vi "Main.vi"() -> ()   [LabVIEW 2020]
uses:
  SET-.ctl
  SET+.ctl
  indicater_CRUI_setpooint.ctl
  I1.ctl
  DIS.ctl
  CRUIONOFF.ctl
  CRUISEVOLUM.ctl
  THONG/STOP.ctl
  CHARDC.ctl
  <vilib>/addons/control/pid/autopid.llb/PID autotuning parameters (adv).ctl
  BRAKE.ctl
  GAS.ctl
  ODOVELICOCITY.ctl
  RPM.ctl
  indicater_dis.ctl
  indicater_Time.ctl
  indicater_taget.ctl
  <vilib>/addons/control/pid/pid.llb/PID Time Unit.ctl
  <vilib>/addons/control/pid/pid.llb/PID Structure.ctl
  <vilib>/addons/control/pid/pid.llb/PID Gain Unit.ctl
  LITMIT.ctl
  SETLIMIT+.ctl
  SETLIMIT-.ctl
  indicater_lit.ctl
  indicater_PWM.ctl
  P.ctl
  R.ctl
  N.ctl
  D.ctl
  CCC.ctl
  <vilib>/Instr/_visa.llb/VISA Configure Serial Port (Instr).vi
  <vilib>/addons/control/pid/pid.llb/PID Structure Conversion (DBL).vi
  <vilib>/addons/control/pid/pid.llb/PID Advanced (DBL).vi
  <vilib>/addons/control/pid/NI_PID_autopid.lvlib
  <vilib>/ptbypt/NI_PtbyPt.lvlib
  <vilib>/addons/control/pid/NI_PID_pid.lvlib
panel:
  out "Waveform Chart 2":T1
  out "D":T2
  out "N":T3
  out "R":T4
  out "P":T5=TRUE
  out "PWM Previous":T6
  in  "auto? ACC":bool
  out "Limit Setpoint":T7
  out "Limit Active":bool
  in  "Limit -":T8
  in  "Limit +":T9
  in  "Limit Speed":T10
  in  "gamma":dbl format="%.2f"
  in  "alpha":dbl=0.2 format="%.2f"
  in  "CHARDC.ctlproportional unit":T11 items=["Gain (K)", "Band (PB)"]
  in  "PID structure":T12 items=["Academic (Standard)", "Parallel", "Series"]
  in  "derivative unit":T13=1 items=["min", "s"]
  in  "integral unit":T13=1 items=["min", "s"]
  in  "derivative":dbl
  in  "integral":dbl
  in  "proportional":dbl=10.0
  in  "linearity":dbl=0.9 format="%.2f"
  in  "beta":dbl=0.7 format="%.2f"
  in  "reinitialize? (F) 2":bool
  out "Speed Setpoint (km/h)":dbl
  out "Target Distance (m)":T14
  out "Time Level":T15=1
  out "Distance (m)":T16=53
  out "Brake Light":bool
  in  "VISA resource name":refnum<visa-resource-name>="COM15"
  in  "baud rate":u32=115200
  out "RPM":T17 scale=0.0..650.0
  out "VELOCITY":T18 scale=0.0..250.0
  out "GAS PEDAL":T19 scale=0.0..700.0
  out "BRAKE PEDAL":T20=1 scale=0.0..700.0
  in  "autotune? (F)":bool
  in  "PID gains":T21={"proportional gain (Kc)"=0.261831, "integral time (Ti, min)"=0.013639, "derivative time (Td, min)"=0.0} {"derivative time (Td, min)" format="%#.6g"; "integral time (Ti, min)" format="%#.6g"; "proportional gain (Kc)" format="%#.6g"}
  in  "dt (s)":dbl=0.02
  in  "reinitialize? (F)":bool
  in  "autotuning parameters":T22={"technique"=0, "type of controller"=1, "control specification"=0, "amplitude"=30.0} {"amplitude" format="%.2f"; "control specification" items=["normal", "fast", "slow"]; "type of controller" items=["P", "PI", "PID"]; "technique" items=["Step Open Loop", "Step Closed Loop", "Relay", "PID Relay"]}
  out "completed?":bool
  out "tuned PID gains":T23={"proportional gain (Kc)"=0.638776, "CHARDC.ctlintegral time (Ti, min)"=0.011721, "derivative time (Td, min)"=0.0} {"derivative time (Td, min)" format="%#.6g"; "CHARDC.ctlintegral time (Ti, min)" format="%#.6g"; "proportional gain (Kc)" format="%#.6g"}
  in  "auto? Speed Control":bool
  in  "ACCEPT SPEED PID":bool
  out "MOTOR CONTROL":T24
  in  "stop":T25
  in  "PID Mode":T26=1 scale=1.0..3.0
  in  "Cruise Enable":T27
  in  "Distance":T28
  out "Distance Level":T29=1
  out "Cruise Active":bool
  out "Cruise Setpoint":T30
  in  "Speed +":T31
  in  "Speed -":T32
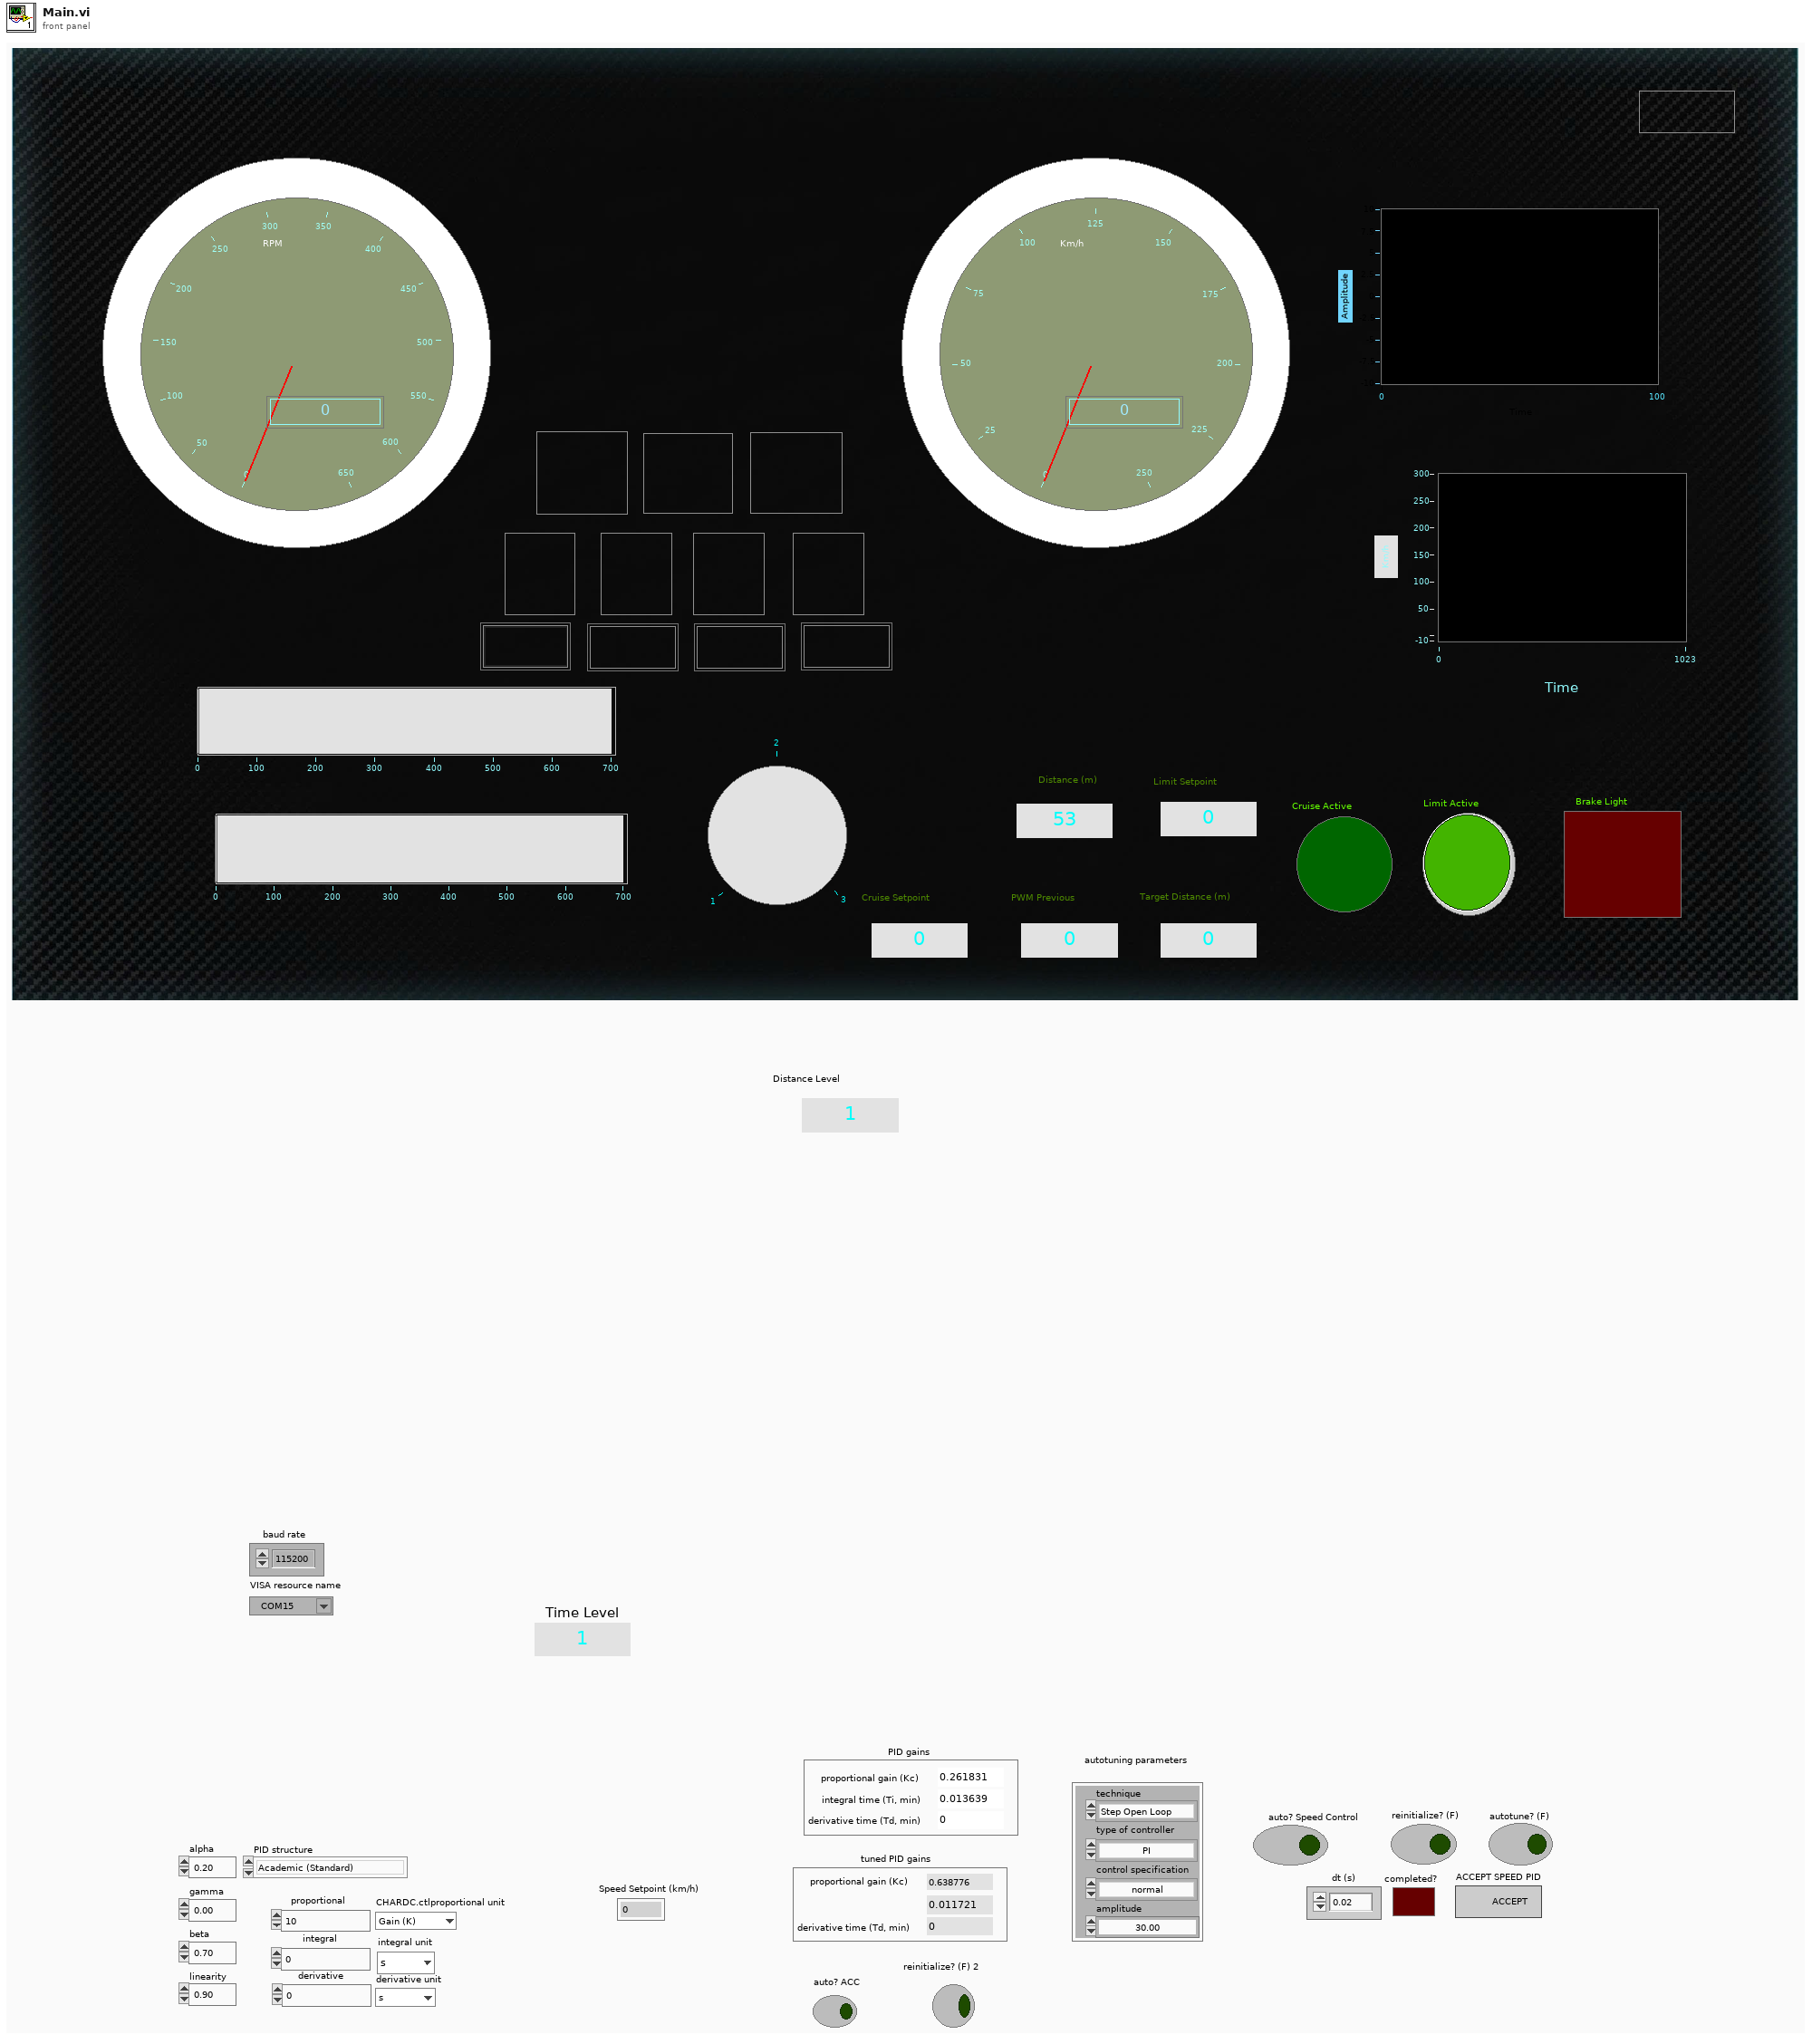
[diagram p1: front panel]
types:
  T1 = typedef "CCC.ctl" = cluster{"VELOCITY":u16, "Cruise Setpoint":u64}
  T2 = typedef "D.ctl" = bool
  T3 = typedef "N.ctl" = bool
  T4 = typedef "R.ctl" = bool
  T5 = typedef "P.ctl" = bool
  T6 = typedef "indicater_PWM.ctl" = i8
  T7 = typedef "indicater_lit.ctl" = i8
  T8 = typedef "SETLIMIT-.ctl" = bool
  T9 = typedef "SETLIMIT+.ctl" = bool
  T10 = typedef "LITMIT.ctl" = bool
  T11 = typedef "NI_PID_pid.lvlib/PID Gain Unit.ctl" = u16
  T12 = typedef "NI_PID_pid.lvlib/PID Structure.ctl" = u16
  T13 = typedef "NI_PID_pid.lvlib/PID Time Unit.ctl" = u16
  T14 = typedef "indicater_taget.ctl" = i8
  T15 = typedef "indicater_Time.ctl" = i8
  T16 = typedef "indicater_dis.ctl" = i8
  T17 = typedef "RPM.ctl" = u16
  T18 = typedef "ODOVELICOCITY.ctl" = u16
  T19 = typedef "GAS.ctl" = u8
  T20 = typedef "BRAKE.ctl" = u8
  T21 = cluster{"proportional gain (Kc)":dbl, "integral time (Ti, min)":dbl, "derivative time (Td, min)":dbl}
  T22 = typedef "NI_PID_autopid.lvlib/PID autotuning parameters (adv).ctl" = cluster{"technique":u16, "type of controller":u16, "control specification":u16, "amplitude":dbl}
  T23 = cluster{"proportional gain (Kc)":dbl, "CHARDC.ctlintegral time (Ti, min)":dbl, "derivative time (Td, min)":dbl}
  T24 = typedef "CHARDC.ctl" = dbl
  T25 = typedef "STOP.ctl" = bool
  T26 = typedef "CRUISEVOLUM.ctl" = u8
  T27 = typedef "CRUIONOFF.ctl" = bool
  T28 = typedef "DIS.ctl" = bool
  T29 = typedef "I1.ctl" = i8
  T30 = typedef "indicater_CRUI_setpooint.ctl" = i8
  T31 = typedef "SET+.ctl" = bool
  T32 = typedef "SET-.ctl" = bool
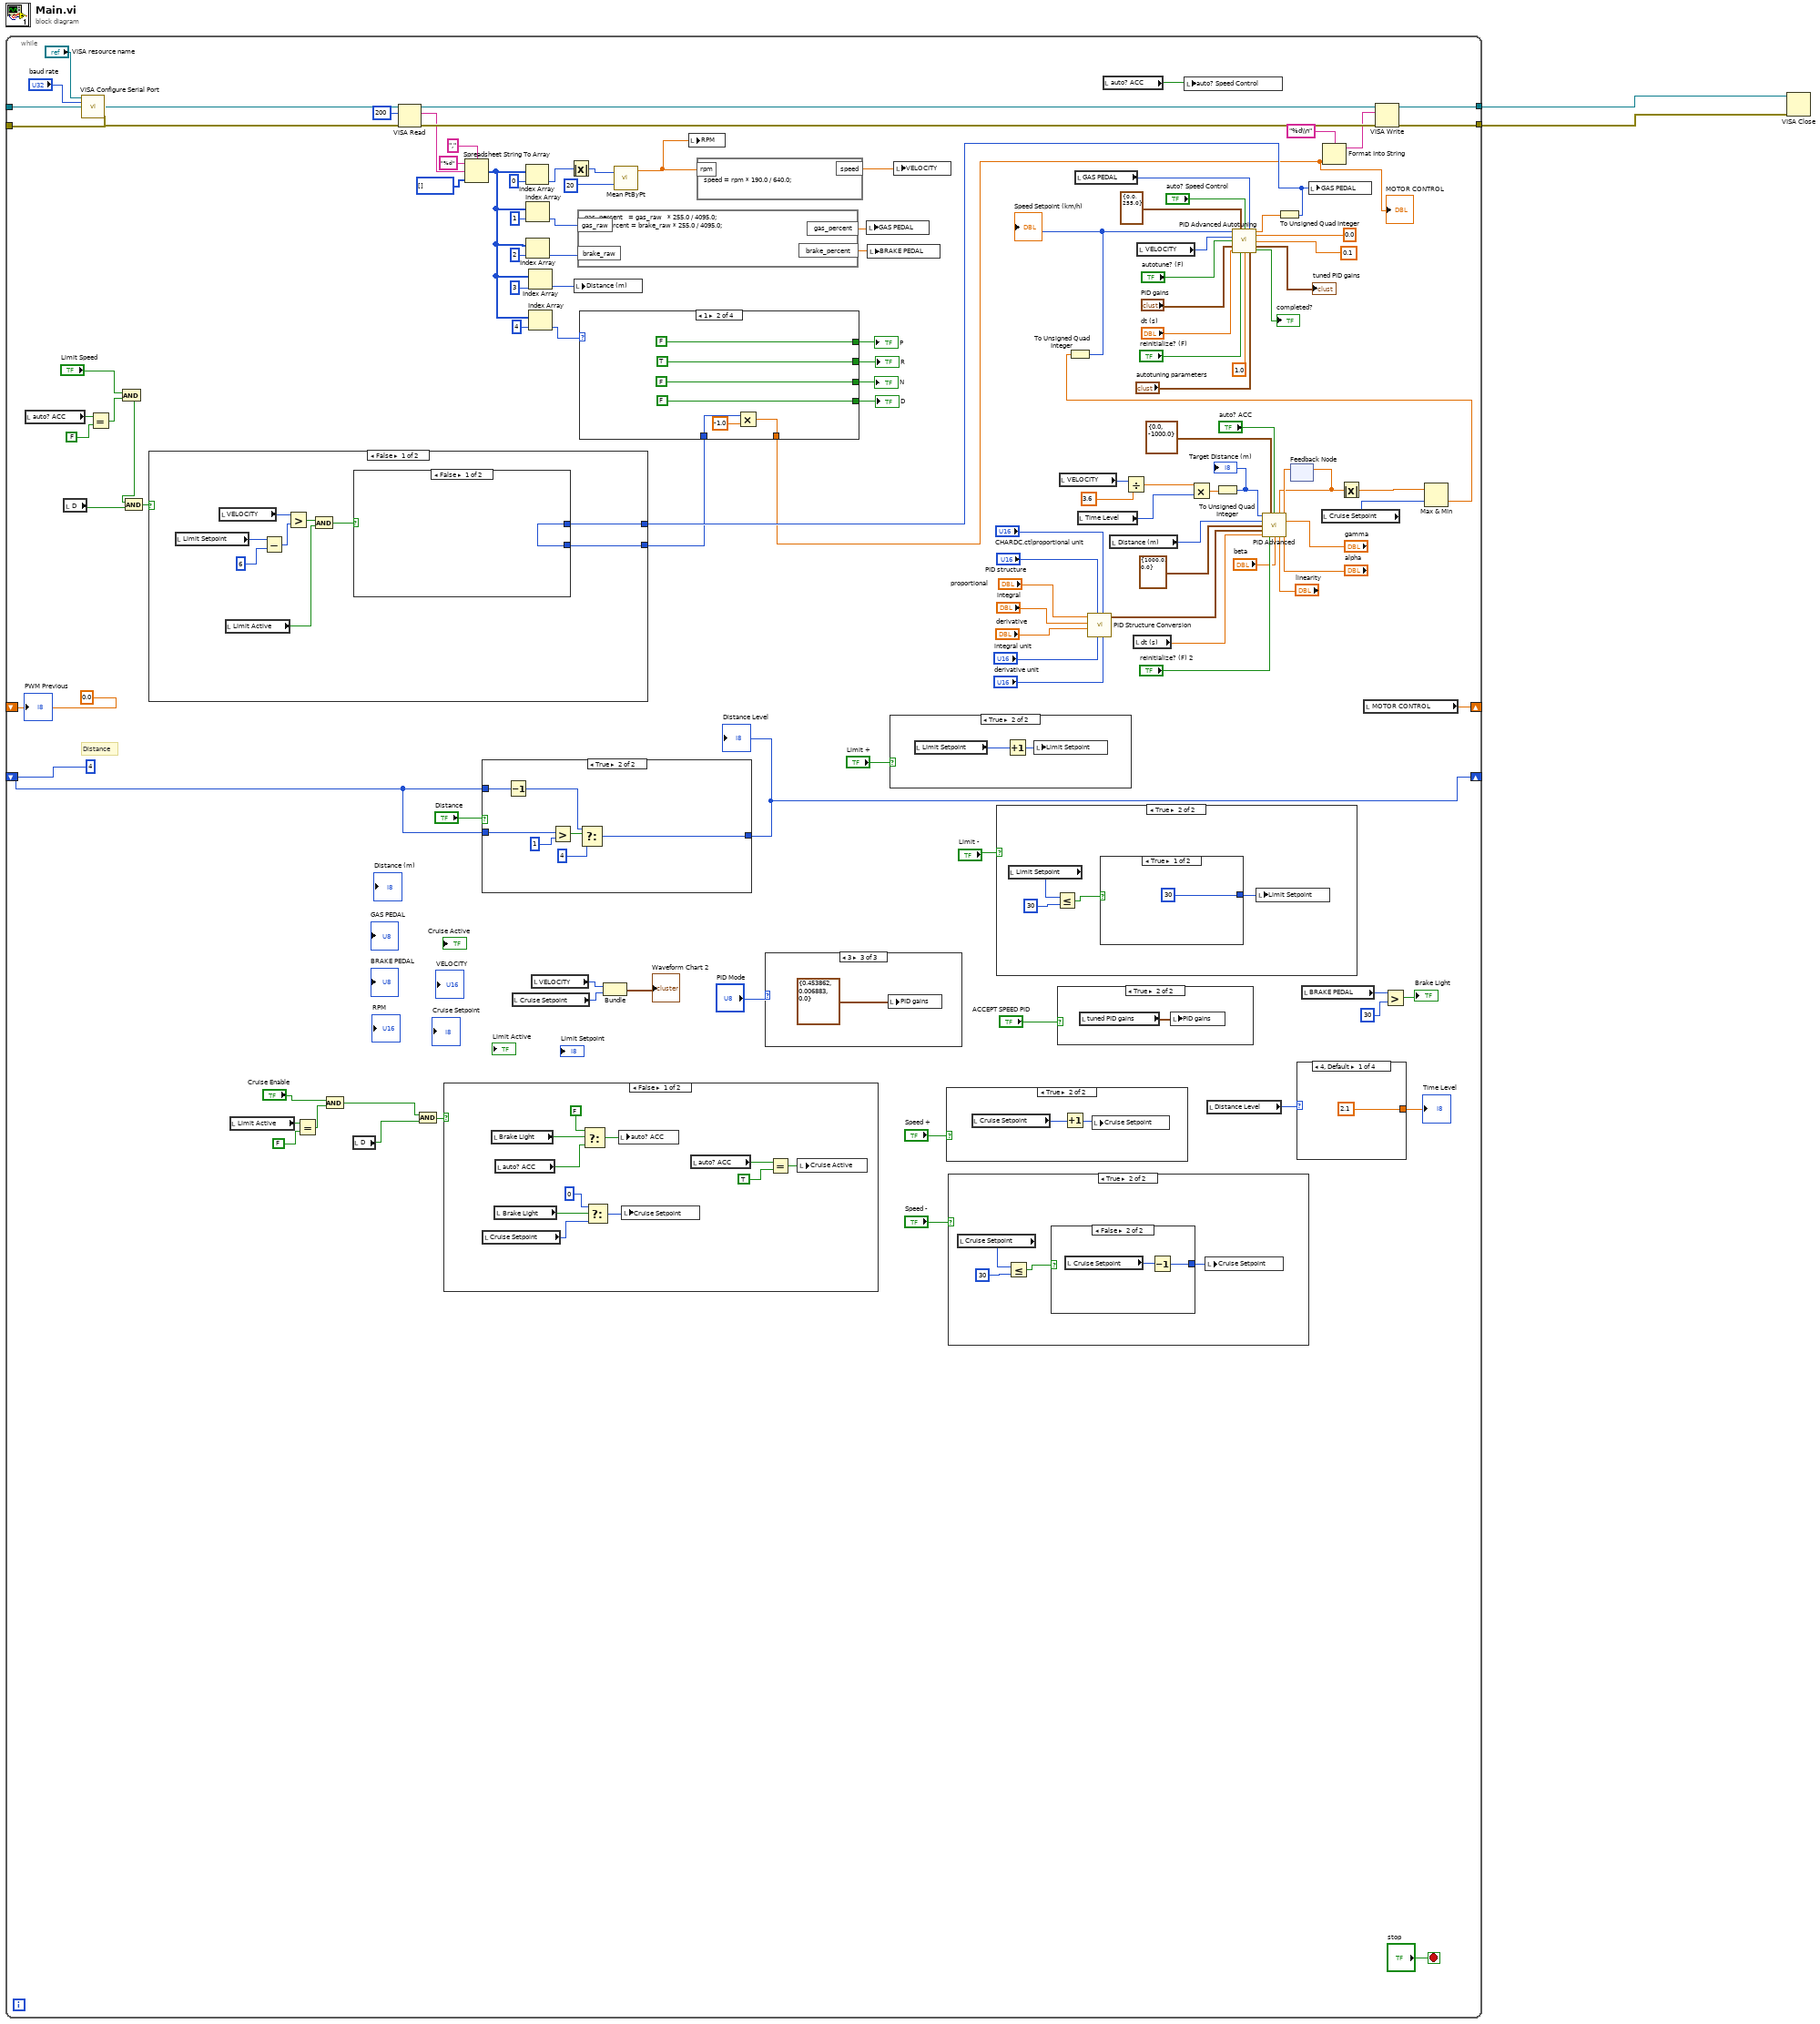
[diagram p0: block diagram]
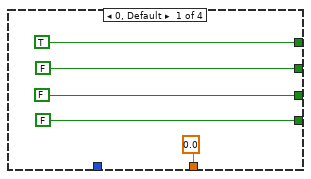
[diagram p2: hidden frame]
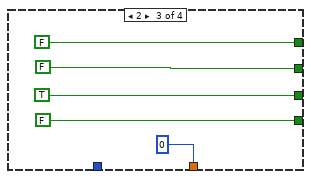
[diagram p3: hidden frame]
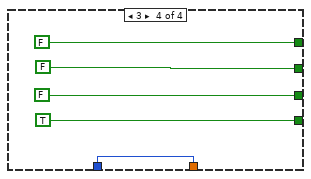
[diagram p4: hidden frame]
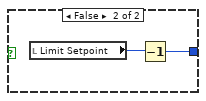
[diagram p6: hidden frame]
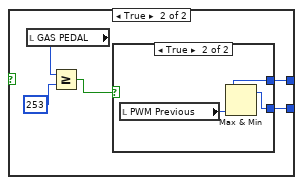
[diagram p8: hidden frame]
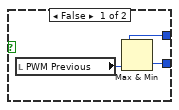
[diagram p9: hidden frame]
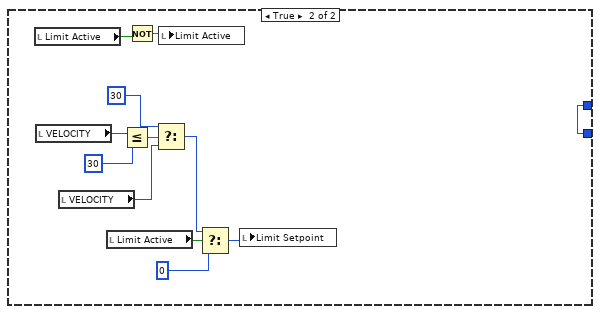
[diagram p10: hidden frame]
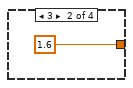
[diagram p11: hidden frame]
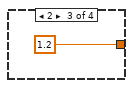
[diagram p12: hidden frame]
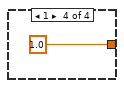
[diagram p13: hidden frame]
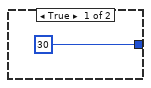
[diagram p16: hidden frame]
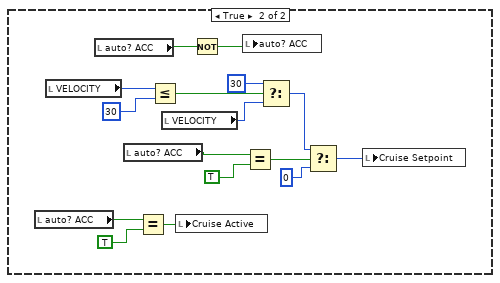
[diagram p18: hidden frame]
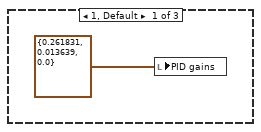
[diagram p19: hidden frame]
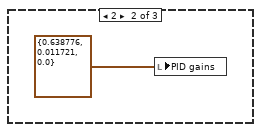
[diagram p20: hidden frame]
diagram:
  # "Distance"
  n1 = call-poly "VISA Configure Serial Port"("VISA resource name"="VISA resource name", "baud rate (9600)"="baud rate") -> ("VISA resource name out"=w7:refnum<visa-resource-name>, "error out"=w6:errorcluster)  [unwired: 12 in]
  n2 = while {
    tunnel: w7 -> [w125]
    tunnel: w6 -> [w124]
    tunnel: [w99] -> w5
    tunnel: [w100] -> w4
    shift-right: [w80] -> _
    shift-left: i64 4 ("f") -> [w81]
    shift-right: [w37] -> _
    shift-left: 0.0 ("MOTOR CONTROL") -> [w35]
    stop <- "stop" stop-if-true
    n3 = local read "auto? ACC"() -> (w41:bool)
    n4 = local read "D"() -> (w17:T2)
    n5 = Equal?(x=w41, y=FALSE) -> (x = y?=w40:bool)
    n6 = And(x="Limit Speed", y=w40) -> (x .and. y?=w18:T10)
    n7 = And(x=w18, y=w17) -> (x .and. y?=w19:T10)
    n8 = local read "Limit Active"() -> (w31:bool)
    n9 = Equal?(x=w31, y=FALSE) -> (x = y?=w32:bool)
    n10 = And(x="Cruise Enable", y=w32) -> (x .and. y?=w15:T27)
    n11 = local read "D"() -> (w14:T2)
    n12 = VISA Read(VISA resource name=w125, byte count=u32 200, error in (no error)=w124) -> (VISA resource name out=w122:refnum<visa-resource-name>, read buffer=w120:string, error out=w123:errorcluster)  [unwired: 1 out]
    n13 = And(x=w15, y=w14) -> (x .and. y?=w16:T27)
    n14 = case shown="False" w16 {
      frame False {
        n15 = local read "Cruise Setpoint"() -> (w213:T30)
        n16 = local read "Brake Light"() -> (w221:bool)
        n17 = local read "Brake Light"() -> (w214:bool)
        n18 = local read "auto? ACC"() -> (w218:bool)
        n19 = Select(t=FALSE, s=w221, f=w218) -> (s? t:f=w219:bool)
        n20 = Select(t=u64 0, s=w214, f=w213) -> (s? t:f=w211:u64)
        n21 = local write "auto? ACC"(w219) -> ()
        n22 = local write "Cruise Setpoint"(w211) -> ()
        n23 = local read "auto? ACC"() -> (w216:bool)
        n24 = Equal?(x=w216, y=TRUE) -> (x = y?=w215:bool)
        n25 = local write "Cruise Active"(w215) -> ()
      }
      frame True {
        n26 = local read "auto? ACC"() -> (w229:bool)
        n27 = local read "VELOCITY"() -> (w228:T18)
        n28 = local read "auto? ACC"() -> (w237:bool)
        n29 = local read "auto? ACC"() -> (w235:bool)
        n30 = Equal?(x=w229, y=TRUE) -> (x = y?=w222:bool)
        n31 = Less Or Equal?(x=w228, y=u64 30) -> (x <= y?=w226:bool)
        n32 = local read "VELOCITY"() -> (w225:T18)
        n33 = local write "Cruise Active"(w222) -> ()
        n34 = Not(x=w237) -> (.not. x?=w236:bool)
        n35 = local write "auto? ACC"(w236) -> ()
        n36 = Equal?(x=w235, y=TRUE) -> (x = y?=w233:bool)
        n37 = Select(t=u64 30, s=w226, f=w225) -> (s? t:f=w223:u64)
        n38 = Select(t=w223, s=w233, f=i64 0) -> (s? t:f=w232:u64)
        n39 = local write "Cruise Setpoint"(w232) -> ()
      }
    }
    n40 = Spreadsheet String To Array(delimiter (Tab)=",", format string="%d", spreadsheet string=w120, array type (2D Dbl)=i32[] []) -> (array=w26:i32[])
    n41 = case shown="True" "Distance" {
      tunnel: w81 -> [w194 w201]
      tunnel: w81 -> [_ w200]
      tunnel: [w194 w195] -> w80
      frame False {
      }
      frame True {
        n42 = Decrement(x=w201) -> (x-1=w197:i64)
        n43 = Greater?(x=w200, y=i64 1) -> (0:w198:bool)
        n44 = Select(t=w197, s=w198, f=i64 4) -> (s? t:f=w195:i64)
      }
    }
    "Distance Level" <- w80
    n45 = local read "Cruise Setpoint"() -> (w10:T30)
    n46 = Index Array(array=w26, index=0) -> (element=w93:i32)
    n47 = Index Array(array=w26, index=1) -> (element=w96:i32)
    n48 = Index Array(array=w26, index=2) -> (element=w95:i32)
    n49 = Index Array(array=w26, index=3) -> (element=w75:i32)
    n50 = Index Array(array=w26, index=4) -> (element=w24:i32)
    n51 = local read "VELOCITY"() -> (w11:T18)
    n52 = Absolute Value(x=w93) -> (abs(x)=w92:i32)
    n53 = local write "Distance (m)"(w75) -> ()
    n54 = formula code="gas_percent   = gas_raw   * 255.0 / 4095.0;\nbrake_percent = brake_raw * 255.0 / 4095.0;"("gas_raw"=w96, "brake_raw"=w95) -> ("gas_percent"=w34:dbl, "brake_percent"=w94:dbl)
    n55 = Bundle("VELOCITY"=w11, "Cruise Setpoint"=w10) -> (→"Waveform Chart 2":cluster{"VELOCITY":T18, "Cruise Setpoint":T30})  [unwired: 1 in]
    n56 = call <vilib>:"Mean PtByPt.vi"("x"=w92, "sample length"=20) -> ("mean"=w97:dbl)  [unwired: 2 in, 1 out]
    n57 = local write "RPM"(w97) -> ()
    n58 = formula code="speed = rpm * 190.0 / 640.0;"("rpm"=w97) -> ("speed"=w98:dbl)
    n59 = case shown="3" "PID Mode" {
      frame 1, Default {
        n60 = local write "PID gains"(T21 {"proportional gain (Kc)"=0.261831, "integral time (Ti, min)"=0.013639, "derivative time (Td, min)"=0.0} ("PID gains")) -> ()
      }
      frame 2 {
        n61 = local write "PID gains"(T21 {"proportional gain (Kc)"=0.638776, "integral time (Ti, min)"=0.011721, "derivative time (Td, min)"=0.0} ("PID gains")) -> ()
      }
      frame 3 {
        n62 = local write "PID gains"(T21 {"proportional gain (Kc)"=0.453862, "integral time (Ti, min)"=0.006883, "derivative time (Td, min)"=0.0} ("PID gains")) -> ()
      }
    }
    n63 = local write "GAS PEDAL"(w34) -> ()
    n64 = local write "BRAKE PEDAL"(w94) -> ()
    n65 = case shown="True" "Limit +" {
      frame False {
      }
      frame True {
        n66 = local read "Limit Setpoint"() -> (w156:T7)
        n67 = Increment(x=w156) -> (x+1=w155:T7)
        n68 = local write "Limit Setpoint"(w155) -> ()
      }
    }
    n69 = local write "VELOCITY"(w98) -> ()
    n70 = case shown="True" "Speed +" {
      frame False {
      }
      frame True {
        n71 = local read "Cruise Setpoint"() -> (w209:T30)
        n72 = Increment(x=w209) -> (x+1=w210:T30)
        n73 = local write "Cruise Setpoint"(w210) -> ()
      }
    }
    n74 = case shown="True" "Speed -" {
      frame False {
      }
      frame True {
        n75 = local read "Cruise Setpoint"() -> (w204:T30)
        n76 = Less Or Equal?(x=w204, y=u64 30) -> (x <= y?=w202:bool)
        n77 = case shown="False" w202 {
          tunnel: [u64 30 ("y") w207] -> w205
          frame True {
          }
          frame False {
            n78 = local read "Cruise Setpoint"() -> (w208:T30)
            n79 = Decrement(x=w208) -> (x-1=w207:T30)
          }
        }
        n80 = local write "Cruise Setpoint"(w205) -> ()
      }
    }
    n81 = case shown="True" "Limit -" {
      frame False {
      }
      frame True {
        n82 = local read "Limit Setpoint"() -> (w150:T7)
        n83 = Less Or Equal?(x=w150, y=u64 30) -> (x <= y?=w148:bool)
        n84 = case shown="True" w148 {
          tunnel: [u64 30 ("y") w153] -> w151
          frame True {
          }
          frame False {
            n85 = local read "Limit Setpoint"() -> (w154:T7)
            n86 = Decrement(x=w154) -> (x-1=w153:T7)
          }
        }
        n87 = local write "Limit Setpoint"(w151) -> ()
      }
    }
    n88 = case shown="True" "ACCEPT SPEED PID" {
      frame False {
      }
      frame True {
        n89 = local read "tuned PID gains"() -> (w241:T23)
        n90 = local write "PID gains"(w241) -> ()
      }
    }
    n91 = local read "VELOCITY"() -> (w69:T18)
    n92 = local read "GAS PEDAL"() -> (w85:T19)
    n93 = local read "Time Level"() -> (w70:T15)
    n94 = call-poly <vilib>:"PID Structure Conversion.vi"("derivative unit"="derivative unit", "proportional unit"="CHARDC.ctlproportional unit", "integral unit"="integral unit", "PID structure"="PID structure", "derivative"="derivative", "integral"="integral", "proportional"="proportional") -> ("PID gains"=w46:T21)  [unwired: 4 in]
    n95 = local read "auto? ACC"() -> (w42:bool)
    n96 = local read "Distance (m)"() -> (w68:T16)
    n97 = Divide(x=w69, y=3.6) -> (x/y=w71:dbl)
    n98 = local read "dt (s)"() -> (w62:dbl)
    n99 = local read "VELOCITY"() -> (w111:T18)
    n100 = local write "auto? Speed Control"(w42) -> ()
    n101 = Multiply(x=w71, y=w70) -> (x*y=w57:dbl)
    n102 = local read "Distance Level"() -> (w74:T29)
    n103 = To Unsigned Quad Integer(1:w57) -> (0:w56:u64)
    "Target Distance (m)" <- w56
    n104 = feedback #1() -> (w61:dbl)  [unwired: 1 in]
    n105 = call-poly <vilib>:"PID Advanced.vi"("setpoint"=w56, "output range"=cluster{"output high":dbl, "output low":dbl} {"output high"=0.0, "output low"=-1000.0}, "auto? (T)"="auto? ACC", "manual control"=w61, "process variable"=w68, "gamma"="gamma", "setpoint range"=cluster{"setpoint high":dbl, "setpoint low":dbl} {"setpoint high"=1000.0, "setpoint low"=0.0}, "alpha"="alpha", "PID gains"=w46, "dt (s)"=w62, "reinitialize? (F)"="reinitialize? (F) 2", "beta"="beta", "linearity"="linearity") -> ("output"=w63:dbl)  [unwired: 1 in, 1 out]
    n106 = feedback-in #1(w63) -> ()
    n107 = case shown="4, Default" w74 {
      tunnel: [2.1 ("Time Level") 1.6 ("Time Level") 1.2 ("Time Level") 1.0 ("Time Level")] -> w73
      frame 4, Default {
      }
      frame 3 {
      }
      frame 2 {
      }
      frame 1 {
      }
    }
    "Time Level" <- w73
    n108 = local read "BRAKE PEDAL"() -> (w79:T20)
    n109 = local read "Cruise Setpoint"() -> (w65:T30)
    n110 = Absolute Value(x=w61) -> (abs(x)=w60:dbl)
    n111 = local read "MOTOR CONTROL"() -> (w37:T24)
    n112 = Greater?(x=w79, y=u8 30) -> (0:→"Brake Light":bool)
    n113 = Max & Min(x=w60, y=w65) -> (min(x,y)=w54:dbl)  [unwired: 1 out]
    n114 = To Unsigned Quad Integer(1:w54) -> (0:w55:u64)
    "Speed Setpoint (km/h)" <- w55
    n115 = call <vilib>:"PID Advanced Autotuning.vi"("setpoint"=w55, "output range"=cluster{"output high":dbl, "output low":dbl} {"output high"=0.0, "output low"=255.0}, "auto? (F)"="auto? Speed Control", "manual control"=w85, "process variable"=w111, "gamma"=0.0, "autotune? (F)"="autotune? (F)", "alpha"=0.1, "PID gains"="PID gains", "dt (s)"="dt (s)", "reinitialize? (F)"="reinitialize? (F)", "beta"=1.0, "autotuning parameters"="autotuning parameters") -> ("output"=w28:dbl, "tuned PID gains"=→"tuned PID gains":T21, "tuning completed?"=→"completed?":bool)
    n116 = To Unsigned Quad Integer(1:w28) -> (0:w27:u64)
    n117 = case shown="False" w19 {
      tunnel: w27 -> [w164 w178]
      tunnel: [w163 w178] -> w13
      frame False {
        n118 = local read "Limit Setpoint"() -> (w158:T7)
        n119 = local read "VELOCITY"() -> (w165:T18)
        n120 = local read "Limit Active"() -> (w161:bool)
        n121 = Subtract(x=w158, y=u64 6) -> (x-y=w159:u64)
        n122 = Greater?(x=w165, y=w159) -> (0:w162:bool)
        n123 = And(x=w162, y=w161) -> (x .and. y?=w160:bool)
        n124 = case shown="False" w160 {
          tunnel: w164 -> [w166 w171]
          tunnel: [w166 w170] -> w163
          frame False {
          }
          frame True {
            n125 = local read "GAS PEDAL"() -> (w169:T19)
            n126 = Greater Or Equal?(x=w169, y=u8 253) -> (x >= y?=w167:bool)
            n127 = case shown="True" w167 {
              tunnel: w171 -> [w173 w176]
              tunnel: [w172 w175] -> w170
              frame False {
                n128 = local read "PWM Previous"() -> (w174:T6)
                n129 = Max & Min(x=w173, y=w174) -> (min(x,y)=w172:u64)  [unwired: 1 out]
              }
              frame True {
                n130 = local read "PWM Previous"() -> (w177:T6)
                n131 = Max & Min(x=w176, y=w177) -> (max(x,y)=w175:u64)  [unwired: 1 out]
              }
            }
          }
        }
      }
      frame True {
        n132 = local read "Limit Active"() -> (w183:bool)
        n133 = local read "VELOCITY"() -> (w189:T18)
        n134 = local read "VELOCITY"() -> (w186:T18)
        n135 = local read "Limit Active"() -> (w182:bool)
        n136 = Less Or Equal?(x=w189, y=u64 30) -> (x <= y?=w187:bool)
        n137 = Not(x=w183) -> (.not. x?=w184:bool)
        n138 = Select(t=u64 30, s=w187, f=w186) -> (s? t:f=w181:u64)
        n139 = local write "Limit Active"(w184) -> ()
        n140 = Select(t=w181, s=w182, f=u64 0) -> (s? t:f=w179:u64)
        n141 = local write "Limit Setpoint"(w179) -> ()
      }
    }
    n142 = case shown="1" w24 {
      tunnel: [FALSE ("D") FALSE ("D") FALSE ("D") TRUE ("D")] -> w23
      tunnel: [FALSE ("N") FALSE ("N") TRUE ("N") FALSE ("N")] -> w22
      tunnel: [FALSE ("R") TRUE ("R") FALSE ("R") FALSE ("R")] -> w21
      tunnel: [TRUE ("P") FALSE ("P") FALSE ("P") FALSE ("P")] -> w20
      tunnel: w13 -> [_ w133 _ w143]
      tunnel: [0.0 ("index") w132 0 ("index") w143] -> w12
      frame 0, Default {
      }
      frame 1 {
        n143 = Multiply(x=w133, y=-1.0) -> (x*y=w132:dbl)
      }
      frame 2 {
      }
      frame 3 {
      }
    }
    "MOTOR CONTROL" <- w12
    "P" <- w20
    "R" <- w21
    "N" <- w22
    "D" <- w23
    n144 = local write "GAS PEDAL"(w27) -> ()
    n145 = Format Into String(format string="%d\\n", w12) -> (resulting string=w112:string)  [unwired: 2 in, 1 out]
    n146 = VISA Write(VISA resource name=w122, write buffer=w112, error in (no error)=w123) -> (VISA resource name out=w100:refnum<visa-resource-name>, error out=w99:errorcluster)  [unwired: 1 out]
    "PWM Previous" <- w35
  }
  n147 = VISA Close(VISA resource name=w4, error in (no error)=w5) -> ()  [unwired: 1 out]
